vi "Dresden R2R Sputter 03.02.2018 IY24.vi"() -> ()   [LabVIEW 2009] (continued)
                                }
                                }
                                n12390 = case shown="False" w19089 {
                                tunnel: [FALSE TRUE] -> w19090
                                frame #0 {
                                n12391 = Wait Until Next ms Multiple(millisecond multiple=u32 200) -> ()  [unwired: 1 out]
                                }
                                frame #1 {
                                }
                                }
                                }
                              }
                              frame #1 {
                              }
                            }
                          }
                          frame #3 {
                            n12392 = local read "Semi"() -> (w19099:bool)
                            n12393 = case shown="False" w19099 {
                              frame #0 {
                                n12394 = local write "CH1_2_trns_0"(TRUE ("CH1_2_trns_0")) -> ()
                                n12395 = Wait (ms)(milliseconds to wait=u32 1000) -> ()  [unwired: 1 out]
                              }
                              frame #1 {
                              }
                            }
                          }
                        }
                      }
                      frame #1 {
                      }
                    }
                  }
                  frame #1 {
                  }
                }
              }
              frame #1 {
              }
            }
          }
          frame #3 {
            # "STARTED UP CH2"
            n12396 = disable-structure shown="Disabled" {
              frame #0 {
                n12397 = local read "Semi"() -> (w19102:bool)
                n12398 = case shown="False" w19102 {
                  frame #0 {
                    n12399 = local read "started_up_ch2"() -> (w19103:bool)
                    n12400 = case shown="False" w19103 {
                      frame #0 {
                        n12401 = stacked-sequence {
                          frame #0 {
                            n12402 = local read "Semi"() -> (w19104:bool)
                            n12403 = case shown="False" w19104 {
                              frame #0 {
                                n12404 = local write "Start_up_ch2"(TRUE ("Start_up_ch2")) -> ()
                              }
                              frame #1 {
                              }
                            }
                          }
                          frame #1 {
                            n12405 = local read "Semi"() -> (w19106:bool)
                            n12406 = case shown="False" w19106 {
                              frame #0 {
                                n12407 = Wait (ms)(milliseconds to wait=u32 18000) -> ()  [unwired: 1 out]
                              }
                              frame #1 {
                              }
                            }
                          }
                          frame #2 {
                            n12408 = local read "Semi"() -> (w19108:bool)
                            n12409 = case shown="False" w19108 {
                              frame #0 {
                                n12410 = while {
                                i -> [w19113]
                                stop <- w19110 stop-if-true
                                n12411 = Greater?(x=w19113, y=90) -> (0:w19111:bool)
                                n12412 = local read "started_up_ch2"() -> (w19109:bool)
                                n12413 = case shown="True" w19111 {
                                frame #0 {
                                }
                                frame #1 {
                                n12414 = local write "Semi"(TRUE ("Semi")) -> ()
                                n12415 = local write "Error Message"("Chamber 2 Pressure is not suitable  \nfor transfer process!\nPlease check connections." ("Error Message")) -> ()
                                }
                                }
                                n12416 = case shown="False" w19109 {
                                tunnel: [FALSE TRUE] -> w19110
                                frame #0 {
                                n12417 = Wait Until Next ms Multiple(millisecond multiple=u32 200) -> ()  [unwired: 1 out]
                                }
                                frame #1 {
                                }
                                }
                                }
                              }
                              frame #1 {
                              }
                            }
                          }
                          frame #3 {
                            n12418 = local read "Semi"() -> (w19119:bool)
                            n12419 = case shown="False" w19119 {
                              frame #0 {
                                n12420 = local write "CH1_2_trns_1"(TRUE ("CH1_2_trns_0")) -> ()
                                n12421 = Wait (ms)(milliseconds to wait=u32 1000) -> ()  [unwired: 1 out]
                              }
                              frame #1 {
                              }
                            }
                          }
                        }
                      }
                      frame #1 {
                      }
                    }
                  }
                  frame #1 {
                  }
                }
              }
              frame #1 {
              }
            }
          }
          frame #4 {
            # "TRNS GV -BP OPEN"
            n12422 = local read "Semi"() -> (w19122:bool)
            n12423 = case shown="False" w19122 {
              frame #0 {
                n12424 = stacked-sequence {
                  frame #0 {
                    n12425 = local read "Semi"() -> (w19123:bool)
                    n12426 = case shown="False" w19123 {
                      frame #0 {
                        n12427 = while {
                          i -> [w19130]
                          stop <- w19125 stop-if-true
                          n12428 = Greater?(x=w19130, y=50) -> (0:w19128:bool)
                          n12429 = local read "Ch2_trns_gv_bp2_di"() -> (w19124:bool)
                          n12430 = case shown="True" w19128 {
                            frame #0 {
                            }
                            frame #1 {
                              n12431 = local write "Semi"(TRUE ("Semi")) -> ()
                              n12432 = local write "Error Message"("Transfer process was cancelled.\nPlease check CH1-Trns-GV connections." ("Error Message")) -> ()
                            }
                          }
                          n12433 = case shown="False" w19124 {
                            tunnel: [FALSE TRUE] -> w19127
                            frame #0 {
                              n12434 = Wait Until Next ms Multiple(millisecond multiple=u32 200) -> ()  [unwired: 1 out]
                              n12435 = local write "Ch2_trns_gv_bp2_do"(TRUE ("Ch1_pet_cool_up_do")) -> ()
                            }
                            frame #1 {
                            }
                          }
                          n12436 = local read "Semi"() -> (w19126:bool)
                          n12437 = Or(x=w19127, y=w19126) -> (x .or. y?=w19125:bool)
                        }
                      }
                      frame #1 {
                      }
                    }
                  }
                  frame #1 {
                    n12438 = local read "Semi"() -> (w19137:bool)
                    n12439 = case shown="False" w19137 {
                      frame #0 {
                        n12440 = Wait (ms)(milliseconds to wait=u32 500) -> ()  [unwired: 1 out]
                      }
                      frame #1 {
                      }
                    }
                  }
                  frame #2 {
                    n12441 = local read "Semi"() -> (w19139:bool)
                    n12442 = case shown="False" w19139 {
                      frame #0 {
                        n12443 = while {
                          i -> [w19146]
                          stop <- w19141 stop-if-true
                          n12444 = Greater?(x=w19146, y=50) -> (0:w19144:bool)
                          n12445 = local read "Ch3_Trns_gv_bp_di"() -> (w19140:bool)
                          n12446 = case shown="True" w19144 {
                            frame #0 {
                            }
                            frame #1 {
                              n12447 = local write "Semi"(TRUE ("Semi")) -> ()
                              n12448 = local write "Error Message"("Transfer process was cancelled.\nPlease check CH1-Trns-GV connections." ("Error Message")) -> ()
                            }
                          }
                          n12449 = case shown="False" w19140 {
                            tunnel: [FALSE TRUE] -> w19143
                            frame #0 {
                              n12450 = local write "Ch3_Trns_gv_bp_do"(TRUE ("Ch1_pet_cool_up_do")) -> ()
                              n12451 = Wait Until Next ms Multiple(millisecond multiple=u32 200) -> ()  [unwired: 1 out]
                            }
                            frame #1 {
                            }
                          }
                          n12452 = local read "Semi"() -> (w19142:bool)
                          n12453 = Or(x=w19143, y=w19142) -> (x .or. y?=w19141:bool)
                        }
                      }
                      frame #1 {
                      }
                    }
                  }
                  frame #3 {
                    n12454 = local read "Semi"() -> (w19153:bool)
                    n12455 = case shown="False" w19153 {
                      frame #0 {
                        n12456 = Wait (ms)(milliseconds to wait=u32 500) -> ()  [unwired: 1 out]
                      }
                      frame #1 {
                      }
                    }
                  }
                }
              }
              frame #1 {
              }
            }
          }
          frame #5 {
            # "TRNS GV OPEN"
            n12457 = local read "Semi"() -> (w19155:bool)
            n12458 = case shown="False" w19155 {
              frame #0 {
                n12459 = stacked-sequence {
                  frame #0 {
                    n12460 = local read "Semi"() -> (w19156:bool)
                    n12461 = case shown="False" w19156 {
                      frame #0 {
                        n12462 = local write "Ch2_Trns_gv_close_do"(FALSE ("Ch1_pet_cool_up_do")) -> ()
                      }
                      frame #1 {
                      }
                    }
                  }
                  frame #1 {
                    n12463 = local read "Semi"() -> (w19158:bool)
                    n12464 = case shown="False" w19158 {
                      frame #0 {
                        n12465 = while {
                          i -> [w19165]
                          stop <- w19160 stop-if-true
                          n12466 = Greater?(x=w19165, y=500) -> (0:w19163:bool)
                          n12467 = local read "Ch2_Trns_gv_open_di"() -> (w19159:bool)
                          n12468 = case shown="True" w19163 {
                            frame #0 {
                            }
                            frame #1 {
                              n12469 = local write "Semi"(TRUE ("Semi")) -> ()
                              n12470 = local write "Error Message"("Transfer process was cancelled.\nPlease check CH1-Trns-GV connections." ("Error Message")) -> ()
                            }
                          }
                          n12471 = case shown="False" w19159 {
                            tunnel: [FALSE TRUE] -> w19162
                            frame #0 {
                              n12472 = Wait Until Next ms Multiple(millisecond multiple=u32 200) -> ()  [unwired: 1 out]
                              n12473 = local write "Ch2_Trns_gv_open_do"(TRUE ("Ch1_pet_cool_up_do")) -> ()
                            }
                            frame #1 {
                            }
                          }
                          n12474 = local read "Semi"() -> (w19161:bool)
                          n12475 = Or(x=w19162, y=w19161) -> (x .or. y?=w19160:bool)
                        }
                      }
                      frame #1 {
                      }
                    }
                  }
                  frame #2 {
                    n12476 = local read "Semi"() -> (w19172:bool)
                    n12477 = case shown="False" w19172 {
                      frame #0 {
                        n12478 = local write "CH1_2trns_2"(TRUE ("CH1_2trns_5")) -> ()
                        n12479 = Wait (ms)(milliseconds to wait=u32 500) -> ()  [unwired: 1 out]
                      }
                      frame #1 {
                      }
                    }
                  }
                }
              }
              frame #1 {
              }
            }
          }
          frame #6 {
            # "TRNS GV control Trnsgv 2_3"
            n12480 = local read "Semi"() -> (w19175:bool)
            n12481 = case shown="False" w19175 {
              frame #0 {
                n12482 = stacked-sequence {
                  frame #0 {
                    n12483 = local read "Semi"() -> (w19176:bool)
                    n12484 = case shown="False" w19176 {
                      frame #0 {
                        n12485 = while {
                          i -> [w19183]
                          stop <- w19178 stop-if-true
                          n12486 = Greater?(x=w19183, y=50) -> (0:w19181:bool)
                          n12487 = local read "Ch2_TGV_control_di"() -> (w19177:bool)
                          n12488 = case shown="True" w19181 {
                            frame #0 {
                            }
                            frame #1 {
                              n12489 = local write "Semi"(TRUE ("Semi")) -> ()
                              n12490 = local write "Error Message"("Transfer process was cancelled.\nPlease check TRNS-GV connections." ("Error Message")) -> ()
                            }
                          }
                          n12491 = case shown="True" w19177 {
                            tunnel: [TRUE FALSE] -> w19180
                            frame #0 {
                            }
                            frame #1 {
                              n12492 = Wait Until Next ms Multiple(millisecond multiple=u32 200) -> ()  [unwired: 1 out]
                              n12493 = local write "Ch2_TGV_control_do"(FALSE ("Ch1_pet_cool_up_do")) -> ()
                            }
                          }
                          n12494 = local read "Semi"() -> (w19179:bool)
                          n12495 = Or(x=w19180, y=w19179) -> (x .or. y?=w19178:bool)
                        }
                      }
                      frame #1 {
                      }
                    }
                  }
                  frame #1 {
                    n12496 = local read "Semi"() -> (w19190:bool)
                    n12497 = case shown="False" w19190 {
                      frame #0 {
                        n12498 = local write "CH1_2trns_3"(TRUE ("CH1_2trns_5")) -> ()
                        n12499 = Wait (ms)(milliseconds to wait=u32 500) -> ()  [unwired: 1 out]
                      }
                      frame #1 {
                      }
                    }
                  }
                }
              }
              frame #1 {
              }
            }
          }
          frame #7 {
            # "TRNS GV control Trnsgv 2_3"
            n12500 = local read "Semi"() -> (w19193:bool)
            n12501 = case shown="False" w19193 {
              frame #0 {
                n12502 = stacked-sequence {
                  frame #0 {
                    n12503 = local read "Semi"() -> (w19194:bool)
                    n12504 = case shown="False" w19194 {
                      frame #0 {
                        n12505 = while {
                          i -> [w19201]
                          stop <- w19196 stop-if-true
                          n12506 = Greater?(x=w19201, y=50) -> (0:w19199:bool)
                          n12507 = local read "Ch1_Trns_interlock_di"() -> (w19195:bool)
                          n12508 = case shown="True" w19199 {
                            frame #0 {
                            }
                            frame #1 {
                              n12509 = local write "Semi"(TRUE ("Semi")) -> ()
                              n12510 = local write "Error Message"("Transfer process was cancelled.\nPlease check TRNS-GV connections." ("Error Message")) -> ()
                            }
                          }
                          n12511 = case shown="False" w19195 {
                            tunnel: [w19203 TRUE] -> w19198
                            frame #0 {
                              n12512 = local read "Ch1_TGV_control_di"() -> (w19202:bool)
                              n12513 = case shown="False" w19202 {
                                tunnel: [FALSE TRUE] -> w19203
                                frame #0 {
                                n12514 = Wait Until Next ms Multiple(millisecond multiple=u32 200) -> ()  [unwired: 1 out]
                                n12515 = local write "Ch1_TGV_control_do"(TRUE ("Ch1_pet_cool_up_do")) -> ()
                                }
                                frame #1 {
                                }
                              }
                            }
                            frame #1 {
                            }
                          }
                          n12516 = local read "Semi"() -> (w19197:bool)
                          n12517 = Or(x=w19198, y=w19197) -> (x .or. y?=w19196:bool)
                        }
                      }
                      frame #1 {
                      }
                    }
                  }
                  frame #1 {
                    n12518 = local read "Semi"() -> (w19211:bool)
                    n12519 = case shown="False" w19211 {
                      frame #0 {
                        n12520 = local write "CH1_2trns_3"(TRUE ("CH1_2trns_5")) -> ()
                        n12521 = Wait (ms)(milliseconds to wait=u32 500) -> ()  [unwired: 1 out]
                      }
                      frame #1 {
                      }
                    }
                  }
                }
              }
              frame #1 {
              }
            }
          }
          frame #8 {
            # "TRNS GV control Trnsgv 3_4"
            n12522 = local read "Semi"() -> (w19214:bool)
            n12523 = case shown="False" w19214 {
              frame #0 {
                n12524 = stacked-sequence {
                  frame #0 {
                    n12525 = local read "Semi"() -> (w19215:bool)
                    n12526 = case shown="False" w19215 {
                      frame #0 {
                        n12527 = while {
                          i -> [w19222]
                          stop <- w19217 stop-if-true
                          n12528 = Greater?(x=w19222, y=50) -> (0:w19220:bool)
                          n12529 = local read "Ch3_Trns_interlock_di"() -> (w19216:bool)
                          n12530 = case shown="True" w19220 {
                            frame #0 {
                            }
                            frame #1 {
                              n12531 = local write "Semi"(TRUE ("Semi")) -> ()
                              n12532 = local write "Error Message"("Transfer process was cancelled.\nPlease check TRNS-GV connections." ("Error Message")) -> ()
                            }
                          }
                          n12533 = case shown="False" w19216 {
                            tunnel: [w19224 TRUE] -> w19219
                            frame #0 {
                              n12534 = local read "Ch3_TGV_control_di"() -> (w19223:bool)
                              n12535 = case shown="False" w19223 {
                                tunnel: [FALSE TRUE] -> w19224
                                frame #0 {
                                n12536 = Wait Until Next ms Multiple(millisecond multiple=u32 200) -> ()  [unwired: 1 out]
                                n12537 = local write "Ch3_TGV_control_do"(TRUE ("Ch1_pet_cool_up_do")) -> ()
                                }
                                frame #1 {
                                }
                              }
                            }
                            frame #1 {
                            }
                          }
                          n12538 = local read "Semi"() -> (w19218:bool)
                          n12539 = Or(x=w19219, y=w19218) -> (x .or. y?=w19217:bool)
                        }
                      }
                      frame #1 {
                      }
                    }
                  }
                  frame #1 {
                    n12540 = local read "Semi"() -> (w19232:bool)
                    n12541 = case shown="False" w19232 {
                      frame #0 {
                        n12542 = local write "CH1_2trns_4"(TRUE ("CH1_2trns_5")) -> ()
                        n12543 = Wait (ms)(milliseconds to wait=u32 500) -> ()  [unwired: 1 out]
                      }
                      frame #1 {
                      }
                    }
                  }
                }
              }
              frame #1 {
              }
            }
          }
          frame #9 {
            # "Right slow deactive"
            n12544 = local read "Semi"() -> (w19235:bool)
            n12545 = case shown="False" w19235 {
              frame #0 {
                n12546 = stacked-sequence {
                  frame #0 {
                    n12547 = local read "Semi"() -> (w19236:bool)
                    n12548 = case shown="False" w19236 {
                      frame #0 {
                        n12549 = while {
                          i -> [w19239]
                          stop <- w19240 stop-if-true
                          n12550 = Greater?(x=w19239, y=50) -> (0:w19237:bool)
                          n12551 = local read "Cnt_Right_slow_di"() -> (w19243:bool)
                          n12552 = case shown="True" w19237 {
                            frame #0 {
                            }
                            frame #1 {
                              n12553 = local write "Semi"(TRUE ("Semi")) -> ()
                              n12554 = local write "Error Message"("Transfer process was\ncancelled.Please check right slow sensor." ("Error Message")) -> ()
                            }
                          }
                          n12555 = case shown="False" w19243 {
                            tunnel: [FALSE ("Ch1_pet_cool_up_do") TRUE ("Ch1_pet_cool_up_do")] -> w19242
                            frame #0 {
                              n12556 = Wait Until Next ms Multiple(millisecond multiple=u32 200) -> ()  [unwired: 1 out]
                              n12557 = local write "Cnt_Right_slow_do"(TRUE ("Ch1_pet_cool_up_do")) -> ()
                            }
                            frame #1 {
                            }
                          }
                          n12558 = local read "Semi"() -> (w19241:bool)
                          n12559 = Or(x=w19242, y=w19241) -> (x .or. y?=w19240:bool)
                        }
                      }
                      frame #1 {
                      }
                    }
                  }
                  frame #1 {
                    n12560 = local read "Semi"() -> (w19250:bool)
                    n12561 = case shown="False" w19250 {
                      frame #0 {
                        n12562 = local write "CH1_2trns_5"(TRUE ("CH1_2trns_7")) -> ()
                        n12563 = Wait (ms)(milliseconds to wait=u32 500) -> ()  [unwired: 1 out]
                      }
                      frame #1 {
                      }
                    }
                  }
                }
              }
              frame #1 {
              }
            }
          }
          frame #10 {
            # "Right limit deactive"
            n12564 = local read "Semi"() -> (w19253:bool)
            n12565 = case shown="False" w19253 {
              frame #0 {
                n12566 = stacked-sequence {
                  frame #0 {
                    n12567 = local read "Semi"() -> (w19254:bool)
                    n12568 = case shown="False" w19254 {
                      frame #0 {
                        n12569 = while {
                          i -> [w19255]
                          stop <- w19259 stop-if-true
                          n12570 = Greater?(x=w19255, y=50) -> (0:w19257:bool)
                          n12571 = local read "Cnt_Right_limit_di"() -> (w19261:bool)
                          n12572 = case shown="True" w19257 {
                            frame #0 {
                            }
                            frame #1 {
                              n12573 = local write "Semi"(TRUE ("Semi")) -> ()
                              n12574 = local write "Error Message"("Transfer process was\ncancelled.Please check right limit sensor." ("Error Message")) -> ()
                            }
                          }
                          n12575 = case shown="False" w19261 {
                            tunnel: [FALSE ("Ch1_pet_cool_up_do") TRUE ("Ch1_pet_cool_up_do")] -> w19260
                            frame #0 {
                              n12576 = Wait Until Next ms Multiple(millisecond multiple=u32 200) -> ()  [unwired: 1 out]
                              n12577 = local write "Cnt_Right_limit_do"(TRUE ("Ch1_pet_cool_up_do")) -> ()
                            }
                            frame #1 {
                            }
                          }
                          n12578 = local read "Semi"() -> (w19258:bool)
                          n12579 = Or(x=w19260, y=w19258) -> (x .or. y?=w19259:bool)
                        }
                      }
                      frame #1 {
                      }
                    }
                  }
                  frame #1 {
                    n12580 = local read "Semi"() -> (w19268:bool)
                    n12581 = case shown="False" w19268 {
                      frame #0 {
                        n12582 = local write "CH1_2trns_6"(TRUE ("CH1_2trns_7")) -> ()
                        n12583 = Wait (ms)(milliseconds to wait=u32 500) -> ()  [unwired: 1 out]
                      }
                      frame #1 {
                      }
                    }
                  }
                }
              }
              frame #1 {
              }
            }
          }
          frame #11 {
            # "Left slow deactive"
            n12584 = local read "Semi"() -> (w19271:bool)
            n12585 = case shown="False" w19271 {
              frame #0 {
                n12586 = stacked-sequence {
                  frame #0 {
                    n12587 = local read "Semi"() -> (w19272:bool)
                    n12588 = case shown="False" w19272 {
                      frame #0 {
                        n12589 = while {
                          i -> [w19273]
                          stop <- w19277 stop-if-true
                          n12590 = Greater?(x=w19273, y=50) -> (0:w19275:bool)
                          n12591 = local read "Cnt_Left_slow_di"() -> (w19279:bool)
                          n12592 = case shown="True" w19275 {
                            frame #0 {
                            }
                            frame #1 {
                              n12593 = local write "Semi"(TRUE ("Semi")) -> ()
                              n12594 = local write "Error Message"("Transfer process was\ncancelled.Please check left slow sensor." ("Error Message")) -> ()
                            }
                          }
                          n12595 = case shown="False" w19279 {
                            tunnel: [FALSE ("Ch1_pet_cool_up_do") TRUE ("Ch1_pet_cool_up_do")] -> w19278
                            frame #0 {
                              n12596 = Wait Until Next ms Multiple(millisecond multiple=u32 200) -> ()  [unwired: 1 out]
                              n12597 = local write "Cnt_Left_slow_do"(TRUE ("Ch1_pet_cool_up_do")) -> ()
                            }
                            frame #1 {
                            }
                          }
                          n12598 = local read "Semi"() -> (w19276:bool)
                          n12599 = Or(x=w19278, y=w19276) -> (x .or. y?=w19277:bool)
                        }
                      }
                      frame #1 {
                      }
                    }
                  }
                  frame #1 {
                    n12600 = local read "Semi"() -> (w19286:bool)
                    n12601 = case shown="False" w19286 {
                      frame #0 {
                        n12602 = local write "CH1_2trns_7"(TRUE ("CH1_2trns_6b")) -> ()
                        n12603 = Wait (ms)(milliseconds to wait=u32 500) -> ()  [unwired: 1 out]
                      }
                      frame #1 {
                      }
                    }
                  }
                }
              }
              frame #1 {
              }
            }
          }
          frame #12 {
            # "Left limit deactive"
            n12604 = local read "Semi"() -> (w19289:bool)
            n12605 = case shown="False" w19289 {
              frame #0 {
                n12606 = stacked-sequence {
                  frame #0 {
                    n12607 = local read "Semi"() -> (w19290:bool)
                    n12608 = case shown="False" w19290 {
                      frame #0 {
                        n12609 = while {
                          i -> [w19291]
                          stop <- w19295 stop-if-true
                          n12610 = Greater?(x=w19291, y=50) -> (0:w19293:bool)
                          n12611 = local read "Cnt_Left_limit_di"() -> (w19297:bool)
                          n12612 = case shown="True" w19293 {
                            frame #0 {
                            }
                            frame #1 {
                              n12613 = local write "Semi"(TRUE ("Semi")) -> ()
                              n12614 = local write "Error Message"("Transfer process was\ncancelled.Please check left limit sensor." ("Error Message")) -> ()
                            }
                          }
                          n12615 = case shown="False" w19297 {
                            tunnel: [FALSE ("Ch1_pet_cool_up_do") TRUE ("Ch1_pet_cool_up_do")] -> w19296
                            frame #0 {
                              n12616 = Wait Until Next ms Multiple(millisecond multiple=u32 200) -> ()  [unwired: 1 out]
                              n12617 = local write "Cnt_Left_limit_do"(TRUE ("Ch1_pet_cool_up_do")) -> ()
                            }
                            frame #1 {
                            }
                          }
                          n12618 = local read "Semi"() -> (w19294:bool)
                          n12619 = Or(x=w19296, y=w19294) -> (x .or. y?=w19295:bool)
                        }
                      }
                      frame #1 {
                      }
                    }
                  }
                  frame #1 {
                    n12620 = local read "Semi"() -> (w19304:bool)
                    n12621 = case shown="False" w19304 {
                      frame #0 {
                        n12622 = local write "CH1_2trns_8"(TRUE ("CH1_2trns_6c")) -> ()
                        n12623 = Wait (ms)(milliseconds to wait=u32 500) -> ()  [unwired: 1 out]
                      }
                      frame #1 {
                      }
                    }
                  }
                }
              }
              frame #1 {
              }
            }
          }
          frame #13 {
            # "Casette Direction"
            n12624 = local read "Semi"() -> (w19307:bool)
            n12625 = case shown="False" w19307 {
              frame #0 {
                n12626 = stacked-sequence {
                  frame #0 {
                    n12627 = local read "Semi"() -> (w19308:bool)
                    n12628 = case shown="False" w19308 {
                      frame #0 {
                        n12629 = while {
                          i -> [w19314]
                          stop <- w19309 stop-if-true
                          n12630 = Greater?(x=w19314, y=50) -> (0:w19315:bool)
                          n12631 = case shown="True" w19315 {
                            frame #0 {
                            }
                            frame #1 {
                              n12632 = local write "Semi"(TRUE ("Semi")) -> ()
                              n12633 = local write "Error Message"("Transfer process was cancelled.\nPlease check Casette Direction connections." ("Error Message")) -> ()
                            }
                          }
                          n12634 = local read "Casette_servo_left_direction_di"() -> (w19312:bool)
                          n12635 = case shown="False" w19312 {
                            tunnel: [FALSE ("Casette_servo_left_direction_do") TRUE ("Casette_servo_left_direction_do")] -> w19311
                            frame #0 {
                              n12636 = Wait Until Next ms Multiple(millisecond multiple=u32 200) -> ()  [unwired: 1 out]
                              n12637 = local write "Casette_servo_left_direction_do"(TRUE ("Casette_servo_left_direction_do")) -> ()
                            }
                            frame #1 {
                            }
                          }
                          n12638 = local read "Semi"() -> (w19310:bool)
                          n12639 = Or(x=w19311, y=w19310) -> (x .or. y?=w19309:bool)
                        }
                      }
                      frame #1 {
                      }
                    }
                  }
                  frame #1 {
                    n12640 = local read "Semi"() -> (w19322:bool)
                    n12641 = case shown="False" w19322 {
                      frame #0 {
                        n12642 = local write "CH1_2trns_9"(TRUE ("CH1_2trns_7")) -> ()
                        n12643 = Wait (ms)(milliseconds to wait=u32 500) -> ()  [unwired: 1 out]
                      }
                      frame #1 {
                      }
                    }
                  }
                }
              }
              frame #1 {
              }
            }
          }
          frame #14 {
            # "SET CASSETTE SERVO  SPEED 300"
            n12644 = local read "Semi"() -> (w19325:bool)
            n12645 = case shown="False" w19325 {
              frame #0 {
                n12646 = stacked-sequence {
                  frame #0 {
                    n12647 = local read "Semi"() -> (w19326:bool)
                    n12648 = case shown="False" w19326 {
                      frame #0 {
                        n12649 = local write "Cassette_servo_speed_value"(u16 300 ("Cassette_servo_speed_value")) -> ()
                      }
                      frame #1 {
                      }
                    }
                  }
                  frame #1 {
                    n12650 = local read "Semi"() -> (w19328:bool)
                    n12651 = case shown="False" w19328 {
                      frame #0 {
                        n12652 = Wait (ms)(milliseconds to wait=u32 200) -> ()  [unwired: 1 out]
                      }
                      frame #1 {
                      }
                    }
                  }
                  frame #2 {
                    n12653 = local read "Semi"() -> (w19330:bool)
                    n12654 = case shown="False" w19330 {
                      frame #0 {
                        n12655 = local write "Cassette_servo_speed_auto_set"(TRUE ("Cassette_servo_speed_set")) -> ()
                      }
                      frame #1 {
                      }
                    }
                  }
                  frame #3 {
                    n12656 = local read "Semi"() -> (w19332:bool)
                    n12657 = case shown="False" w19332 {
                      frame #0 {
                        n12658 = Wait (ms)(milliseconds to wait=u32 200) -> ()  [unwired: 1 out]
                      }
                      frame #1 {
                      }
                    }
                  }
                  frame #4 {
                    n12659 = local read "Semi"() -> (w19334:bool)
                    n12660 = case shown="False" w19334 {
                      frame #0 {
                        n12661 = local write "CH1_2trns_10"(TRUE ("CH1_2trns_7")) -> ()
                        n12662 = Wait (ms)(milliseconds to wait=u32 500) -> ()  [unwired: 1 out]
                      }
                      frame #1 {
                      }
                    }
                  }
                }
              }
              frame #1 {
              }
            }
          }
          frame #15 {
            # "Casette Servo Start"
            n12663 = local read "Semi"() -> (w19337:bool)
            n12664 = case shown="False" w19337 {
              frame #0 {
                n12665 = stacked-sequence {
                  frame #0 {
                    n12666 = while {
                      i -> [w19343]
                      stop <- w19338 stop-if-true
                      n12667 = Greater?(x=w19343, y=50) -> (0:w19344:bool)
                      n12668 = local read "Casette_servo_start/stop_di"() -> (w19341:bool)
                      n12669 = case shown="True" w19344 {
                        frame #0 {
                        }
                        frame #1 {
                          n12670 = local write "Semi"(TRUE ("Semi")) -> ()
                          n12671 = local write "Error Message"("Transfer process was cancelled.\nPlease check Casette connections." ("Error Message")) -> ()
                        }
                      }
                      n12672 = case shown="False" w19341 {
                        tunnel: [FALSE ("Casette_servo_left_direction_do") TRUE ("Casette_servo_left_direction_do")] -> w19340
                        frame #0 {
                          n12673 = Wait Until Next ms Multiple(millisecond multiple=u32 200) -> ()  [unwired: 1 out]
                          n12674 = local write "Casette_servo_start/stop_do"(TRUE ("Casette_servo_left_direction_do")) -> ()
                        }
                        frame #1 {
                        }
                      }
                      n12675 = local read "Semi"() -> (w19339:bool)
                      n12676 = Or(x=w19340, y=w19339) -> (x .or. y?=w19338:bool)
                    }
                  }
                  frame #1 {
                    n12677 = local read "Semi"() -> (w19351:bool)
                    n12678 = case shown="False" w19351 {
                      frame #0 {
                        n12679 = local write "CH1_2trns_11"(TRUE ("CH1_2trns_9")) -> ()
                        n12680 = Wait (ms)(milliseconds to wait=u32 500) -> ()  [unwired: 1 out]
                      }
                      frame #1 {
                      }
                    }
                  }
                }
              }
              frame #1 {
              }
            }
          }
          frame #16 {
            # "Left sensors activate"
            n12681 = local read "Semi"() -> (w19354:bool)
            n12682 = case shown="False" w19354 {
              frame #0 {
                n12683 = stacked-sequence {
                  frame #0 {
                    n12684 = while {
                      i -> [w19363]
                      stop <- w19359 stop-if-true
                      n12685 = local read "Counter_read_data"() -> (w19356:i16)
                      n12686 = Greater?(x=w19363, y=1500) -> (0:w19362:bool)
                      n12687 = case shown="True" w19362 {
                        frame #0 {
                        }
                        frame #1 {
                          n12688 = local write "Semi"(TRUE ("Semi")) -> ()
                          n12689 = local write "Error Message"("Transfer process was cancelled.\nPlease check Casette & Sensor\nconnections." ("Error Message")) -> ()
                        }
                      }
                      n12690 = Greater Or Equal?(x=w19356, y=i16 3580) -> (x >= y?=w19357:bool)
                      n12691 = case shown="True" w19357 {
                        tunnel: [FALSE TRUE] -> w19360
                        frame #0 {
                          n12692 = Wait Until Next ms Multiple(millisecond multiple=u32 200) -> ()  [unwired: 1 out]
                        }
                        frame #1 {
                        }
                      }
                      n12693 = local read "Semi"() -> (w19358:bool)
                      n12694 = Or(x=w19360, y=w19358) -> (x .or. y?=w19359:bool)
                    }
                  }
                  frame #1 {
                    n12695 = while {
                      i -> [w19372]
                      stop <- w19369 stop-if-true
                      n12696 = Greater?(x=w19372, y=50) -> (0:w19373:bool)
                      n12697 = local read "Cnt_Left_slow_di"() -> (w19375:bool)
                      n12698 = case shown="True" w19373 {
                        frame #0 {
                        }
                        frame #1 {
                          n12699 = local write "Semi"(TRUE ("Semi")) -> ()
                          n12700 = local write "Error Message"("\nPlease check Left Slow Sensor\nconnections." ("Error Message")) -> ()
                        }
                      }
                      n12701 = case shown="True" w19375 {
                        tunnel: [TRUE ("Cnt_Left_slow_do") FALSE ("Cnt_Left_slow_do")] -> w19371
                        frame #0 {
                        }
                        frame #1 {
                          n12702 = Wait Until Next ms Multiple(millisecond multiple=u32 200) -> ()  [unwired: 1 out]
                          n12703 = local write "Cnt_Left_slow_do"(FALSE ("Cnt_Left_slow_do")) -> ()
                        }
                      }
                      n12704 = local read "Semi"() -> (w19370:bool)
                      n12705 = Or(x=w19371, y=w19370) -> (x .or. y?=w19369:bool)
                    }
                  }
                  frame #2 {
                    n12706 = while {
                      i -> [w19385]
                      stop <- w19382 stop-if-true
                      n12707 = Greater?(x=w19385, y=50) -> (0:w19386:bool)
                      n12708 = local read "Cnt_Left_limit_di"() -> (w19388:bool)
                      n12709 = case shown="True" w19386 {
                        frame #0 {
                        }
                        frame #1 {
                          n12710 = local write "Semi"(TRUE ("Semi")) -> ()
                          n12711 = local write "Error Message"("\nPlease check Left Limit Sensor\n connections." ("Error Message")) -> ()
                        }
                      }
                      n12712 = case shown="True" w19388 {
                        tunnel: [TRUE ("Cnt_Left_slow_do") FALSE ("Cnt_Left_slow_do")] -> w19384
                        frame #0 {
                        }
                        frame #1 {
                          n12713 = Wait Until Next ms Multiple(millisecond multiple=u32 200) -> ()  [unwired: 1 out]
                          n12714 = local write "Cnt_Left_limit_do"(FALSE ("Cnt_Left_slow_do")) -> ()
                        }
                      }
                      n12715 = local read "Semi"() -> (w19383:bool)
                      n12716 = Or(x=w19384, y=w19383) -> (x .or. y?=w19382:bool)
                    }
                  }
                  frame #3 {
                    n12717 = local read "Semi"() -> (w19395:bool)
                    n12718 = case shown="False" w19395 {
                      frame #0 {
                        n12719 = local write "CH1_2trns_12"(TRUE ("CH1_2trns_11")) -> ()
                        n12720 = Wait (ms)(milliseconds to wait=u32 500) -> ()  [unwired: 1 out]
                      }
                      frame #1 {